vi "CRYO_MASTER_FULL_dev.vi"() -> ()   [LabVIEW 2017] (continued)
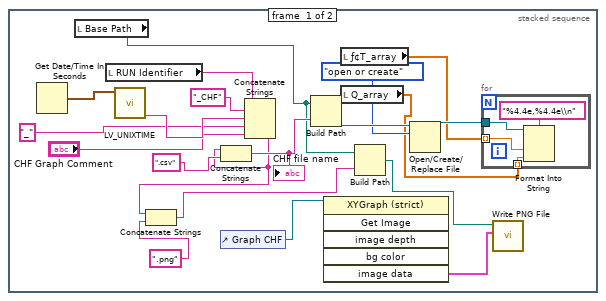
[diagram p3: hidden frame]
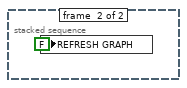
[diagram p5: hidden frame]
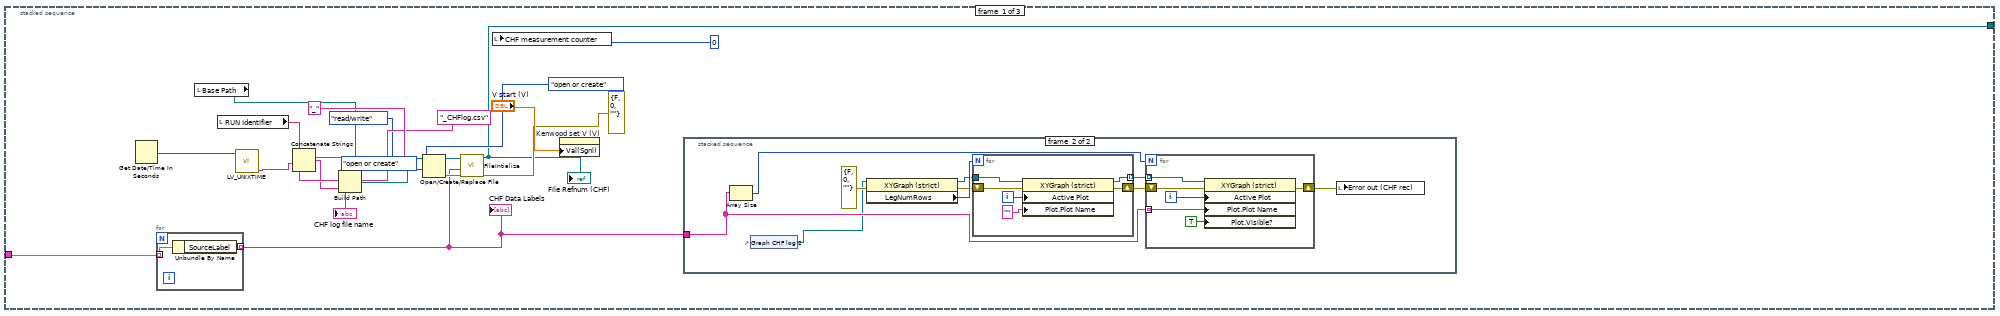
[diagram p7: hidden frame]
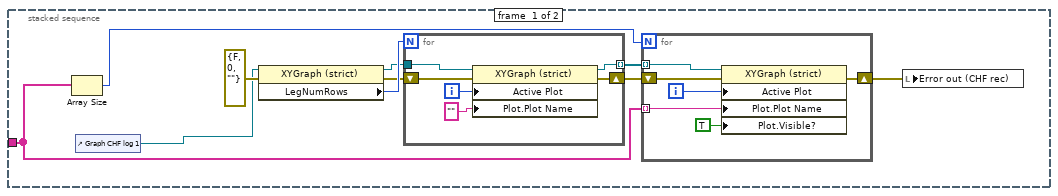
[diagram p8: hidden frame]
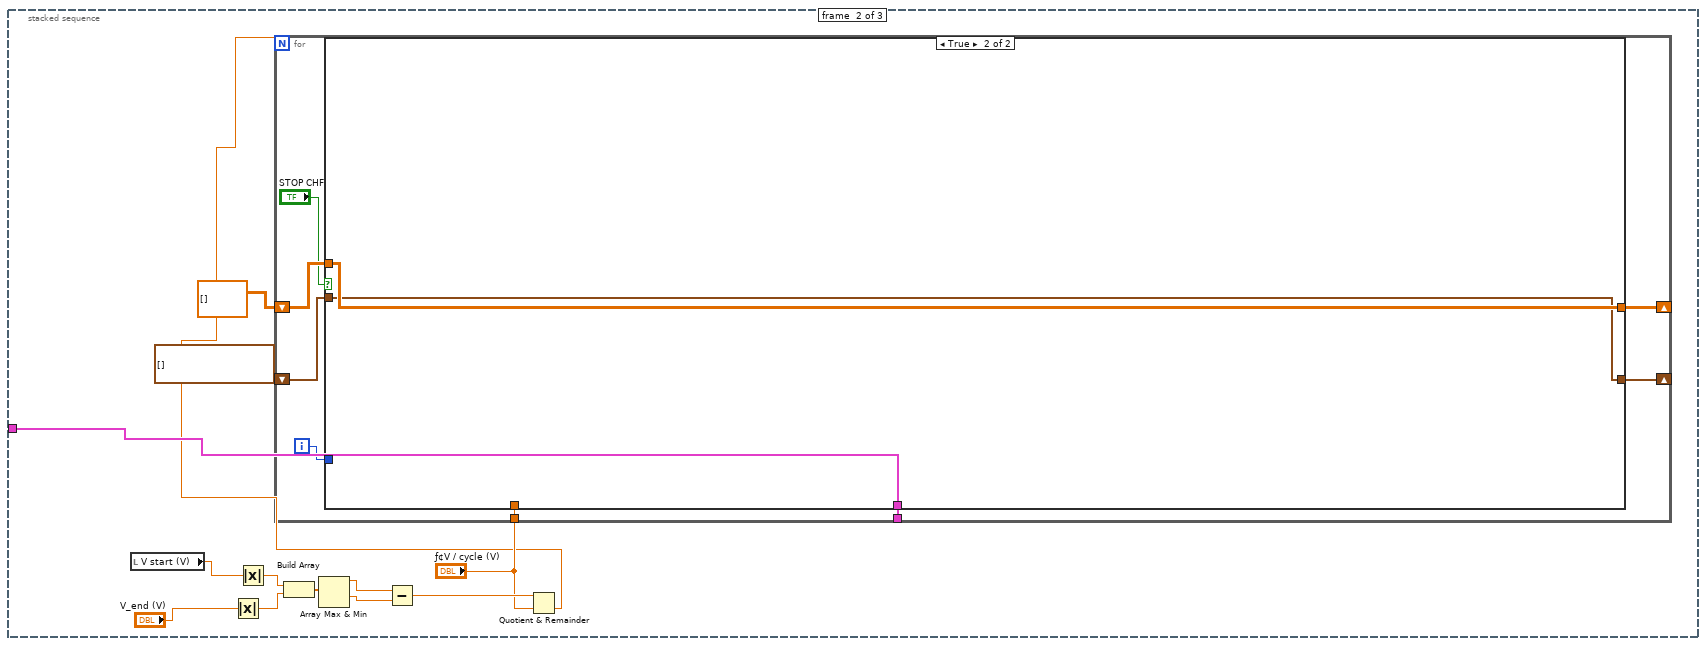
[diagram p9: hidden frame]
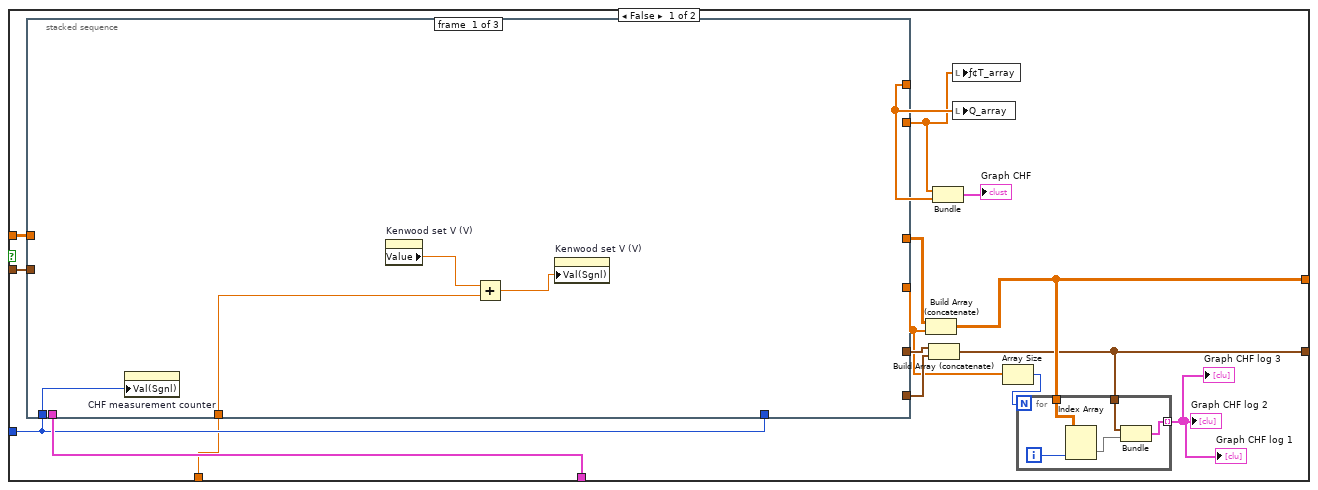
[diagram p10: hidden frame]
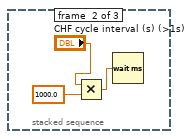
[diagram p11: hidden frame]
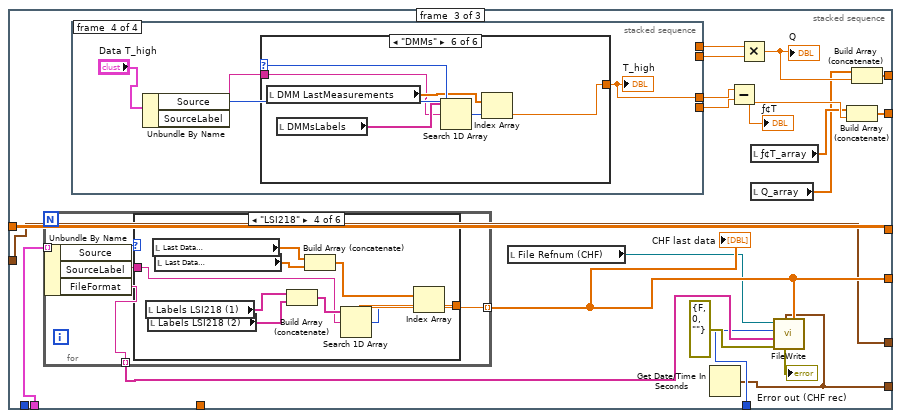
[diagram p12: hidden frame]
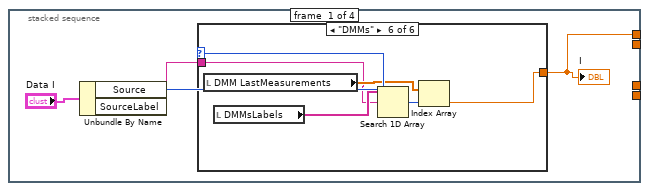
[diagram p13: hidden frame]
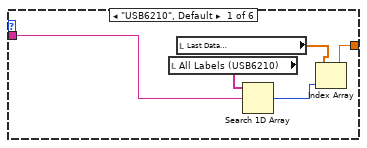
[diagram p14: hidden frame]
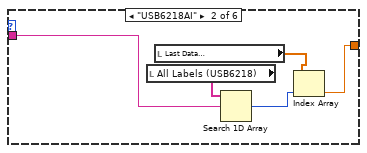
[diagram p15: hidden frame]
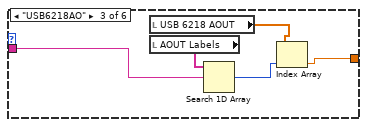
[diagram p16: hidden frame]
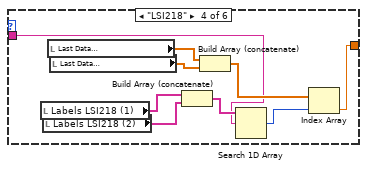
[diagram p17: hidden frame]
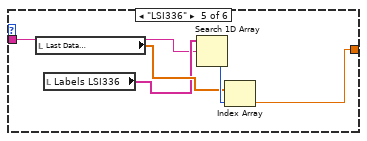
[diagram p18: hidden frame]
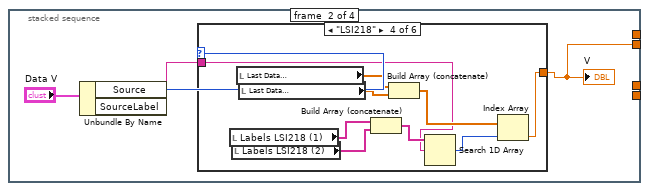
[diagram p19: hidden frame]
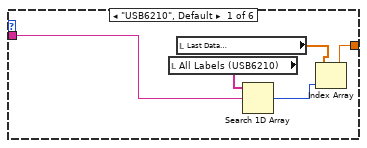
[diagram p20: hidden frame]
    "Cycle #" <- w842
  }
  n1008 = while {
    tunnel: w5 -> [w2128]
    tunnel: w4 -> [w2127]
    stop <- w2129 stop-if-true
    n1009 = Wait (ms)(milliseconds to wait=u32 214) -> ()  [unwired: 1 out]
    n1010 = case shown="True" "RECORD GRAPH" {
      frame False {
      }
      frame True {
        n1011 = stacked-sequence {
          frame #0 {
            n1012 = Get Date/Time In Seconds() -> (seconds since 1Jan1904=w2150:timestamp)
            n1013 = local read "Base Path"() -> (w2135:path)
            n1014 = local read "RUN Identifier"() -> (w2151:string)
            n1015 = call "LV_UNIXTIME.vi"("current time"=w2150) -> ("date/time string"=w2152:string)  [unwired: 9 in, 1 out]
            n1016 = control-ref of="Graph CHF"() -> (w2141:refnum<vi>)
            n1017 = Concatenate Strings(w2151, "_CHF" ("string"), w2152, "_" ("string"), "CHF Graph Comment") -> (w2137:string)
            n1018 = Concatenate Strings(w2137, ".png" ("string")) -> (w2136:string)
            n1019 = Concatenate Strings(w2137, ".csv" ("string")) -> (w2139:string)
            "CHF file name" <- w2139
            n1020 = Build Path(base path=w2135, name or relative path=w2139) -> (appended path=w2146:path)
            n1021 = invoke class="XYGraph (strict)" method="Get Image"(reference=w2141) -> ("image data"=w2133:T23)  [unwired: 5 in, 5 out]
            n1022 = local read "ƒ¢T_array"() -> (w2143:dbl[])
            n1023 = local read "Q_array"() -> (w2142:dbl[])
            n1024 = Build Path(base path=w2135, name or relative path=w2136) -> (appended path=w2134:path)
            n1025 = Open/Create/Replace File(file path (use dialog)=w2146, operation (0:open)=T24."open or create") -> (refnum out=w2144:refnum<file>)  [unwired: 4 in, 2 out]
            n1026 = for {
              tunnel: w2144 -> [w2156]
              tunnel: w2143 -> [w2154] mode=indexing
              tunnel: w2142 -> [w2153] mode=indexing
              n1027 = Format Into String(format string="%4.4e,%4.4e\\n" ("prompt"), initial string=w2156, w2154, w2153) -> ()  [unwired: 1 in, 2 out]
            }
            n1028 = call <vilib>:"Write PNG File.vi"("image data"=w2133, "path to PNG file"=w2134) -> ()  [unwired: 8 in, 2 out]
          }
          frame #1 {
            n1029 = local write "RECORD GRAPH"(FALSE ("RECORD GRAPH")) -> ()
          }
        }
      }
    }
    n1030 = case shown="True" "START CHF" {
      tunnel: "RecordSettings" -> [_ w2161]
      frame False {
      }
      frame True {
        n1031 = stacked-sequence {
          tunnel: [w2165 _ _] -> _
          tunnel: w2161 -> [w2164 w2238 _]
          frame #0 {
            (unwired) T24."open or create" ("operation (0:open)")
            n1032 = Get Date/Time In Seconds() -> (seconds since 1Jan1904=w2177:timestamp)
            n1033 = for {
              tunnel: [w2225] -> w2163 mode=indexing
              tunnel: w2164 -> [w2224] mode=indexing
              n1034 = Unbundle By Name(w2224) -> ("SourceLabel"=w2225:string)
            }
            "CHF Data Labels" <- w2163
            n1035 = local read "Base Path"() -> (w2172:path)
            n1036 = local read "RUN Identifier"() -> (w2176:string)
            n1037 = call "LV_UNIXTIME.vi"("current time"=w2177) -> ("date/time string"=w2175:string)  [unwired: 9 in, 1 out]
            n1038 = Concatenate Strings(w2176, "_" ("string"), w2175, "_CHFlog.csv" ("string")) -> (w2171:string)
            "CHF log file name" <- w2171
            n1039 = Build Path(base path=w2172, name or relative path=w2171) -> (appended path=w2170:path)
            n1040 = Open/Create/Replace File(file path (use dialog)=w2170, error in=errorcluster {"status"=FALSE, "code"=0, "source"=""}, operation (0:open)=T24."open or create", access (0:read/write)=enum16{"read/write", "read-only", "write-only"}."read/write") -> (refnum out=w2168:refnum<file>, error out=w2167:errorcluster)  [unwired: 2 in, 1 out]
            n1041 = call "FileIntialize.vi"("Error In"=w2167, "Labels"=w2163, "refnum in"=w2168) -> ("File Refnum"=w2165:refnum<file>)  [unwired: 7 in, 1 out]
            "File Refnum (CHF)" <- w2165
            n1042 = local write "CHF measurement counter"(0 ("CHF counter")) -> ()
            n1043 = property on="Kenwood set V (V)" class="DigNum (strict)"("Val(Sgnl)"="V start (V)") -> ()  [unwired: 2 in, 2 out]
            n1044 = stacked-sequence {
              tunnel: w2163 -> [w2181 w2204]
              frame #0 {
                n1045 = Array Size(array=w2181) -> (size(s)=w2189:i32)
                n1046 = control-ref of="Graph CHF log 1"() -> (w2182:refnum<vi>)
                n1047 = property class="XYGraph (strict)"(reference=w2182, error in=errorcluster {"status"=FALSE, "code"=0, "source"=""} ("error in (no error)")) -> (reference out=w2184:refnum<vi>, error out=w2186:errorcluster, "LegNumRows"=w2187:u32)
                n1048 = for {
                  N: w2187 -> [_]
                  shift-right: [w2198] -> w2188
                  shift-left: w2186 -> [w2199]
                  tunnel: w2184 -> [w2197]
                  tunnel: [w2196] -> w2183 mode=indexing
                  i -> [w2201]
                  n1049 = property class="XYGraph (strict)"(reference=w2197, error in=w2199, "Active Plot"=w2201, "Plot.Plot Name"="") -> (reference out=w2196:refnum<vi>, error out=w2198:errorcluster)
                }
                n1050 = for {
                  N: w2189 -> [_]
                  shift-right: [w2193] -> w2180
                  shift-left: w2188 -> [w2194]
                  tunnel: w2183 -> [w2191] mode=indexing
                  tunnel: w2181 -> [w2190] mode=indexing
                  i -> [w2195]
                  n1051 = property class="XYGraph (strict)"(reference=w2191, error in=w2194, "Active Plot"=w2195, "Plot.Plot Name"=w2190, "Plot.Visible?"=TRUE ("Plot.Visible")) -> (error out=w2193:errorcluster)  [unwired: 1 out]
                }
                n1052 = local write "Error out (CHF rec)"(w2180) -> ()
              }
              frame #1 {
                n1053 = Array Size(array=w2204) -> (size(s)=w2211:i32)
                n1054 = control-ref of="Graph CHF log 2"() -> (w2203:refnum<vi>)
                n1055 = property class="XYGraph (strict)"(reference=w2203, error in=errorcluster {"status"=FALSE, "code"=0, "source"=""} ("error in (no error)")) -> (reference out=w2206:refnum<vi>, error out=w2208:errorcluster, "LegNumRows"=w2209:u32)
                n1056 = for {
                  N: w2209 -> [_]
                  shift-right: [w2220] -> w2210
                  shift-left: w2208 -> [w2221]
                  tunnel: w2206 -> [w2219]
                  tunnel: [w2218] -> w2205 mode=indexing
                  i -> [w2223]
                  n1057 = property class="XYGraph (strict)"(reference=w2219, error in=w2221, "Active Plot"=w2223, "Plot.Plot Name"="") -> (reference out=w2218:refnum<vi>, error out=w2220:errorcluster)
                }
                n1058 = for {
                  N: w2211 -> [_]
                  shift-right: [w2215] -> w2202
                  shift-left: w2210 -> [w2216]
                  tunnel: w2205 -> [w2213] mode=indexing
                  tunnel: w2204 -> [w2212] mode=indexing
                  i -> [w2217]
                  n1059 = property class="XYGraph (strict)"(reference=w2213, error in=w2216, "Active Plot"=w2217, "Plot.Plot Name"=w2212, "Plot.Visible?"=TRUE ("Plot.Visible")) -> (error out=w2215:errorcluster)  [unwired: 1 out]
                }
                n1060 = local write "Error out (CHF rec)"(w2202) -> ()
              }
            }
          }
          frame #1 {
            n1061 = local read "V start (V)"() -> (w2237:dbl)
            n1062 = Absolute Value(x="V_end (V)") -> (abs(x)=w2234:dbl)
            n1063 = Absolute Value(x=w2237) -> (abs(x)=w2235:dbl)
            n1064 = Build Array(w2235, w2234) -> (w2233:dbl[])
            n1065 = Array Max & Min(array=w2233) -> (max value=w2232:dbl, min value=w2231:dbl)  [unwired: 2 out]
            n1066 = Subtract(x=w2232, y=w2231) -> (x-y=w2230:dbl)
            n1067 = Quotient & Remainder(x=w2230, y="ƒ¢V / cycle (V)") -> (floor(x/y)=w2228:dbl)  [unwired: 1 out]
            n1068 = for {
              N: w2228 -> [_]
              tunnel: w2238 -> [w2246]
              shift-right: [w2242] -> _
              shift-left: dbl[][] [] -> [w2244]
              shift-right: [w2241] -> _
              shift-left: timestamp[] [] -> [w2243]
              tunnel: "ƒ¢V / cycle (V)" -> [w2240]
              i -> [w2245]
              n1069 = case shown="True" "STOP CHF" {
                tunnel: w2246 -> [w2262 _]
                tunnel: w2245 -> [w2261 _]
                tunnel: w2244 -> [w2260 w2487]
                tunnel: w2243 -> [w2256 w2486]
                tunnel: [w2253 w2487] -> w2242
                tunnel: [w2252 w2486] -> w2241
                tunnel: w2240 -> [w2247 _]
                frame False {
                  n1070 = stacked-sequence {
                    tunnel: w2262 -> [_ _ w2294]
                    tunnel: [_ _ w2285] -> w2251
                    tunnel: w2261 -> [_ _ w2284]
                    tunnel: w2261 -> [w2269 _ _]
                    tunnel: [_ _ w2282] -> w2250
                    tunnel: [_ _ w2281] -> w2255
                    tunnel: [_ _ w2280] -> w2259
                    tunnel: w2260 -> [_ _ w2280]
                    tunnel: [_ _ w2279] -> w2258
                    tunnel: w2256 -> [_ _ w2278]
                    tunnel: [_ _ w2278] -> w2257
                    tunnel: w2247 -> [w2268 _ _]
                    frame #0 {
                      n1071 = property on="CHF measurement counter" class="DigNum (strict)"("Val(Sgnl)"=w2269) -> ()  [unwired: 2 in, 2 out]
                      n1072 = property on="Kenwood set V (V)" class="DigNum (strict)"() -> ("Value"=w2271:dbl)  [unwired: 2 in, 2 out]
                      n1073 = Add(x=w2271, y=w2268) -> (x+y=w2270:dbl)
                      n1074 = property on="Kenwood set V (V)" class="DigNum (strict)"("Val(Sgnl)"=w2270) -> ()  [unwired: 2 in, 2 out]
                    }
                    frame #1 {
                      n1075 = Multiply(x="CHF cycle interval (s) (>1s)", y=1000.0) -> (x*y=w2273:dbl)
                      n1076 = Wait (ms)(milliseconds to wait=w2273) -> ()  [unwired: 1 out]
                    }
                    frame #2 {
                      n1077 = for {
                        tunnel: w2294 -> [w2451] mode=indexing
                        tunnel: [w2449] -> w2281 mode=indexing
                        tunnel: [w2447] -> w2292 mode=indexing
                        n1078 = Unbundle By Name(w2451) -> ("Source"=w2450:T36, "SourceLabel"=w2448:string, "FileFormat"=w2447:string)
                        n1079 = case shown="\"LSI218\"" w2450 {
                          tunnel: [w2452 w2457 w2462 w2468 w2476 w2481] -> w2449
                          tunnel: w2448 -> [w2453 w2459 w2464 w2467 w2477 w2485]
                          frame "USB6210", Default {
                            n1080 = local read "All Labels (USB6210)"() -> (w2455:string[])
                            n1081 = local read "Last Data \n(USB6210)"() -> (w2456:dbl[])
                            n1082 = Search 1D Array(1D array=w2455, element=w2453) -> (index of element=w2454:i32)  [unwired: 1 in]
                            n1083 = Index Array(array=w2456, index=w2454) -> (element=w2452:dbl)
                          }
                          frame "USB6218AI" {
                            n1084 = local read "All Labels (USB6218)"() -> (w2460:string[])
                            n1085 = local read "Last Data \n(USB6218)"() -> (w2461:dbl[])
                            n1086 = Search 1D Array(1D array=w2460, element=w2459) -> (index of element=w2458:i32)  [unwired: 1 in]
                            n1087 = Index Array(array=w2461, index=w2458) -> (element=w2457:dbl)
                          }
                          frame "USB6218AO" {
                            n1088 = local read "USB 6218 AOUT"() -> (w2466:dbl[])
                            n1089 = local read "AOUT Labels"() -> (w2465:string[])
                            n1090 = Search 1D Array(1D array=w2465, element=w2464) -> (index of element=w2463:i32)  [unwired: 1 in]
                            n1091 = Index Array(array=w2466, index=w2463) -> (element=w2462:dbl)
                          }
                          frame "LSI218" {
                            n1092 = local read "Labels LSI218 (1)"() -> (w2471:string[])
                            n1093 = local read "Labels LSI218 (2)"() -> (w2470:string[])
                            n1094 = local read "Last Data \nLSI218 (1)"() -> (w2474:dbl[])
                            n1095 = local read "Last Data \nLSI218 (2)"() -> (w2473:dbl[])
                            n1096 = Build Array (concatenate)(w2471, w2470) -> (w2469:string[])
                            n1097 = Build Array (concatenate)(w2474, w2473) -> (w2472:dbl[])
                            n1098 = Search 1D Array(1D array=w2469, element=w2467) -> (index of element=w2475:i32)  [unwired: 1 in]
                            n1099 = Index Array(array=w2472, index=w2475) -> (element=w2468:dbl)
                          }
                          frame "LSI336" {
                            n1100 = local read "Last Data \nLSI336"() -> (w2479:dbl[])
                            n1101 = local read "Labels LSI336"() -> (w2480:string[])
                            n1102 = Search 1D Array(1D array=w2480, element=w2477) -> (index of element=w2478:i32)  [unwired: 1 in]
                            n1103 = Index Array(array=w2479, index=w2478) -> (element=w2476:dbl)
                          }
                          frame "DMMs" {
                            n1104 = local read "DMM LastMeasurements"() -> (w2482:dbl[])
                            n1105 = local read "DMMsLabels"() -> (w2484:string[])
                            n1106 = Search 1D Array(1D array=w2484, element=w2485) -> (index of element=w2483:i32)  [unwired: 1 in]
                            n1107 = Index Array(array=w2482, index=w2483) -> (element=w2481:dbl)
                          }
                        }
                      }
                      "CHF last data" <- w2281
                      n1108 = stacked-sequence {
                        tunnel: [w2295 _ _ _] -> w2290
                        tunnel: [_ w2333 _ _] -> w2289
                        tunnel: [_ _ _ w2409] -> w2288
                        tunnel: [_ _ w2371 _] -> w2287
                        frame #0 {
                          n1109 = Unbundle By Name("Data I") -> ("Source"=w2297:T36, "SourceLabel"=w2296:string)
                          n1110 = case shown="\"DMMs\"" w2297 {
                            tunnel: w2296 -> [w2300 w2305 w2310 w2315 w2324 w2329]
                            tunnel: [w2299 w2304 w2309 w2314 w2323 w2328] -> w2295
                            frame "USB6210", Default {
                              n1111 = local read "All Labels (USB6210)"() -> (w2302:string[])
                              n1112 = local read "Last Data \n(USB6210)"() -> (w2301:dbl[])
                              n1113 = Search 1D Array(1D array=w2302, element=w2300) -> (index of element=w2303:i32)  [unwired: 1 in]
                              n1114 = Index Array(array=w2301, index=w2303) -> (element=w2299:dbl)
                            }
                            frame "USB6218AI" {
                              n1115 = local read "All Labels (USB6218)"() -> (w2307:string[])
                              n1116 = local read "Last Data \n(USB6218)"() -> (w2306:dbl[])
                              n1117 = Search 1D Array(1D array=w2307, element=w2305) -> (index of element=w2308:i32)  [unwired: 1 in]
                              n1118 = Index Array(array=w2306, index=w2308) -> (element=w2304:dbl)
                            }
                            frame "USB6218AO" {
                              n1119 = local read "USB 6218 AOUT"() -> (w2311:dbl[])
                              n1120 = local read "AOUT Labels"() -> (w2312:string[])
                              n1121 = Search 1D Array(1D array=w2312, element=w2310) -> (index of element=w2313:i32)  [unwired: 1 in]
                              n1122 = Index Array(array=w2311, index=w2313) -> (element=w2309:dbl)
                            }
                            frame "LSI218" {
                              n1123 = local read "Labels LSI218 (1)"() -> (w2320:string[])
                              n1124 = local read "Labels LSI218 (2)"() -> (w2321:string[])
                              n1125 = local read "Last Data \nLSI218 (1)"() -> (w2317:dbl[])
                              n1126 = local read "Last Data \nLSI218 (2)"() -> (w2318:dbl[])
                              n1127 = Build Array (concatenate)(w2320, w2321) -> (w2322:string[])
                              n1128 = Build Array (concatenate)(w2317, w2318) -> (w2319:dbl[])
                              n1129 = Search 1D Array(1D array=w2322, element=w2315) -> (index of element=w2316:i32)  [unwired: 1 in]
                              n1130 = Index Array(array=w2319, index=w2316) -> (element=w2314:dbl)
                            }
                            frame "LSI336" {
                              n1131 = local read "Last Data \nLSI336"() -> (w2326:dbl[])
                              n1132 = local read "Labels LSI336"() -> (w2325:string[])
                              n1133 = Search 1D Array(1D array=w2325, element=w2324) -> (index of element=w2327:i32)  [unwired: 1 in]
                              n1134 = Index Array(array=w2326, index=w2327) -> (element=w2323:dbl)
                            }
                            frame "DMMs" {
                              n1135 = local read "DMM LastMeasurements"() -> (w2332:dbl[])
                              n1136 = local read "DMMsLabels"() -> (w2330:string[])
                              n1137 = Search 1D Array(1D array=w2330, element=w2329) -> (index of element=w2331:i32)  [unwired: 1 in]
                              n1138 = Index Array(array=w2332, index=w2331) -> (element=w2328:dbl)
                            }
                          }
                          "I" <- w2295
                        }
                        frame #1 {
                          n1139 = Unbundle By Name("Data V") -> ("Source"=w2336:T36, "SourceLabel"=w2335:string)
                          n1140 = case shown="\"LSI218\"" w2336 {
                            tunnel: w2335 -> [w2338 w2343 w2348 w2353 w2362 w2367]
                            tunnel: [w2337 w2342 w2347 w2352 w2361 w2366] -> w2333
                            frame "USB6210", Default {
                              n1141 = local read "All Labels (USB6210)"() -> (w2340:string[])
                              n1142 = local read "Last Data \n(USB6210)"() -> (w2339:dbl[])
                              n1143 = Search 1D Array(1D array=w2340, element=w2338) -> (index of element=w2341:i32)  [unwired: 1 in]
                              n1144 = Index Array(array=w2339, index=w2341) -> (element=w2337:dbl)
                            }
                            frame "USB6218AI" {
                              n1145 = local read "All Labels (USB6218)"() -> (w2345:string[])
                              n1146 = local read "Last Data \n(USB6218)"() -> (w2344:dbl[])
                              n1147 = Search 1D Array(1D array=w2345, element=w2343) -> (index of element=w2346:i32)  [unwired: 1 in]
                              n1148 = Index Array(array=w2344, index=w2346) -> (element=w2342:dbl)
                            }
                            frame "USB6218AO" {
                              n1149 = local read "USB 6218 AOUT"() -> (w2349:dbl[])
                              n1150 = local read "AOUT Labels"() -> (w2350:string[])
                              n1151 = Search 1D Array(1D array=w2350, element=w2348) -> (index of element=w2351:i32)  [unwired: 1 in]
                              n1152 = Index Array(array=w2349, index=w2351) -> (element=w2347:dbl)
                            }
                            frame "LSI218" {
                              n1153 = local read "Labels LSI218 (1)"() -> (w2358:string[])
                              n1154 = local read "Labels LSI218 (2)"() -> (w2359:string[])
                              n1155 = local read "Last Data \nLSI218 (1)"() -> (w2355:dbl[])
                              n1156 = local read "Last Data \nLSI218 (2)"() -> (w2356:dbl[])
                              n1157 = Build Array (concatenate)(w2358, w2359) -> (w2360:string[])
                              n1158 = Build Array (concatenate)(w2355, w2356) -> (w2357:dbl[])
                              n1159 = Search 1D Array(1D array=w2360, element=w2353) -> (index of element=w2354:i32)  [unwired: 1 in]
                              n1160 = Index Array(array=w2357, index=w2354) -> (element=w2352:dbl)
                            }
                            frame "LSI336" {
                              n1161 = local read "Last Data \nLSI336"() -> (w2364:dbl[])
                              n1162 = local read "Labels LSI336"() -> (w2363:string[])
                              n1163 = Search 1D Array(1D array=w2363, element=w2362) -> (index of element=w2365:i32)  [unwired: 1 in]
                              n1164 = Index Array(array=w2364, index=w2365) -> (element=w2361:dbl)
                            }
                            frame "DMMs" {
                              n1165 = local read "DMM LastMeasurements"() -> (w2370:dbl[])
                              n1166 = local read "DMMsLabels"() -> (w2368:string[])
                              n1167 = Search 1D Array(1D array=w2368, element=w2367) -> (index of element=w2369:i32)  [unwired: 1 in]
                              n1168 = Index Array(array=w2370, index=w2369) -> (element=w2366:dbl)
                            }
                          }
                          "V" <- w2333
                        }
                        frame #2 {
                          n1169 = Unbundle By Name("Data T_low") -> ("Source"=w2374:T36, "SourceLabel"=w2373:string)
                          n1170 = case shown="\"DMMs\"" w2374 {
                            tunnel: w2373 -> [w2376 w2381 w2386 w2391 w2400 w2405]
                            tunnel: [w2375 w2380 w2385 w2390 w2399 w2404] -> w2371
                            frame "USB6210", Default {
                              n1171 = local read "All Labels (USB6210)"() -> (w2378:string[])
                              n1172 = local read "Last Data \n(USB6210)"() -> (w2377:dbl[])
                              n1173 = Search 1D Array(1D array=w2378, element=w2376) -> (index of element=w2379:i32)  [unwired: 1 in]
                              n1174 = Index Array(array=w2377, index=w2379) -> (element=w2375:dbl)
                            }
                            frame "USB6218AI" {
                              n1175 = local read "All Labels (USB6218)"() -> (w2383:string[])
                              n1176 = local read "Last Data \n(USB6218)"() -> (w2382:dbl[])
                              n1177 = Search 1D Array(1D array=w2383, element=w2381) -> (index of element=w2384:i32)  [unwired: 1 in]
                              n1178 = Index Array(array=w2382, index=w2384) -> (element=w2380:dbl)
                            }
                            frame "USB6218AO" {
                              n1179 = local read "USB 6218 AOUT"() -> (w2387:dbl[])
                              n1180 = local read "AOUT Labels"() -> (w2388:string[])
                              n1181 = Search 1D Array(1D array=w2388, element=w2386) -> (index of element=w2389:i32)  [unwired: 1 in]
                              n1182 = Index Array(array=w2387, index=w2389) -> (element=w2385:dbl)
                            }
                            frame "LSI218" {
                              n1183 = local read "Labels LSI218 (1)"() -> (w2396:string[])
                              n1184 = local read "Labels LSI218 (2)"() -> (w2397:string[])
                              n1185 = local read "Last Data \nLSI218 (1)"() -> (w2393:dbl[])
                              n1186 = local read "Last Data \nLSI218 (2)"() -> (w2394:dbl[])
                              n1187 = Build Array (concatenate)(w2396, w2397) -> (w2398:string[])
                              n1188 = Build Array (concatenate)(w2393, w2394) -> (w2395:dbl[])
                              n1189 = Search 1D Array(1D array=w2398, element=w2391) -> (index of element=w2392:i32)  [unwired: 1 in]
                              n1190 = Index Array(array=w2395, index=w2392) -> (element=w2390:dbl)
                            }
                            frame "LSI336" {
                              n1191 = local read "Last Data \nLSI336"() -> (w2402:dbl[])
                              n1192 = local read "Labels LSI336"() -> (w2401:string[])
                              n1193 = Search 1D Array(1D array=w2401, element=w2400) -> (index of element=w2403:i32)  [unwired: 1 in]
                              n1194 = Index Array(array=w2402, index=w2403) -> (element=w2399:dbl)
                            }
                            frame "DMMs" {
                              n1195 = local read "DMM LastMeasurements"() -> (w2408:dbl[])
                              n1196 = local read "DMMsLabels"() -> (w2406:string[])
                              n1197 = Search 1D Array(1D array=w2406, element=w2405) -> (index of element=w2407:i32)  [unwired: 1 in]
                              n1198 = Index Array(array=w2408, index=w2407) -> (element=w2404:dbl)
                            }
                          }
                          "T_low" <- w2371
                        }
                        frame #3 {
                          n1199 = Unbundle By Name("Data T_high") -> ("Source"=w2412:T36, "SourceLabel"=w2411:string)
                          n1200 = case shown="\"DMMs\"" w2412 {
                            tunnel: w2411 -> [w2414 w2419 w2424 w2429 w2438 w2443]
                            tunnel: [w2413 w2418 w2423 w2428 w2437 w2442] -> w2409
                            frame "USB6210", Default {
                              n1201 = local read "All Labels (USB6210)"() -> (w2416:string[])
                              n1202 = local read "Last Data \n(USB6210)"() -> (w2415:dbl[])
                              n1203 = Search 1D Array(1D array=w2416, element=w2414) -> (index of element=w2417:i32)  [unwired: 1 in]
                              n1204 = Index Array(array=w2415, index=w2417) -> (element=w2413:dbl)
                            }
                            frame "USB6218AI" {
                              n1205 = local read "All Labels (USB6218)"() -> (w2421:string[])
                              n1206 = local read "Last Data \n(USB6218)"() -> (w2420:dbl[])
                              n1207 = Search 1D Array(1D array=w2421, element=w2419) -> (index of element=w2422:i32)  [unwired: 1 in]
                              n1208 = Index Array(array=w2420, index=w2422) -> (element=w2418:dbl)
                            }
                            frame "USB6218AO" {
                              n1209 = local read "USB 6218 AOUT"() -> (w2425:dbl[])
                              n1210 = local read "AOUT Labels"() -> (w2426:string[])
                              n1211 = Search 1D Array(1D array=w2426, element=w2424) -> (index of element=w2427:i32)  [unwired: 1 in]
                              n1212 = Index Array(array=w2425, index=w2427) -> (element=w2423:dbl)
                            }
                            frame "LSI218" {
                              n1213 = local read "Labels LSI218 (1)"() -> (w2434:string[])
                              n1214 = local read "Labels LSI218 (2)"() -> (w2435:string[])
                              n1215 = local read "Last Data \nLSI218 (1)"() -> (w2431:dbl[])
                              n1216 = local read "Last Data \nLSI218 (2)"() -> (w2432:dbl[])
                              n1217 = Build Array (concatenate)(w2434, w2435) -> (w2436:string[])
                              n1218 = Build Array (concatenate)(w2431, w2432) -> (w2433:dbl[])
                              n1219 = Search 1D Array(1D array=w2436, element=w2429) -> (index of element=w2430:i32)  [unwired: 1 in]
                              n1220 = Index Array(array=w2433, index=w2430) -> (element=w2428:dbl)
                            }
                            frame "LSI336" {
                              n1221 = local read "Last Data \nLSI336"() -> (w2440:dbl[])
                              n1222 = local read "Labels LSI336"() -> (w2439:string[])
                              n1223 = Search 1D Array(1D array=w2439, element=w2438) -> (index of element=w2441:i32)  [unwired: 1 in]
                              n1224 = Index Array(array=w2440, index=w2441) -> (element=w2437:dbl)
                            }
                            frame "DMMs" {
                              n1225 = local read "DMM LastMeasurements"() -> (w2446:dbl[])
                              n1226 = local read "DMMsLabels"() -> (w2444:string[])
                              n1227 = Search 1D Array(1D array=w2444, element=w2443) -> (index of element=w2445:i32)  [unwired: 1 in]
                              n1228 = Index Array(array=w2446, index=w2445) -> (element=w2442:dbl)
                            }
                          }
                          "T_high" <- w2409
                        }
                      }
                      n1229 = local read "File Refnum (CHF)"() -> (w2275:refnum<file>)
                      n1230 = Get Date/Time In Seconds() -> (seconds since 1Jan1904=w2279:timestamp)
                      n1231 = Subtract(x=w2288, y=w2287) -> (x-y=w2283:dbl)
                      "ƒ¢T" <- w2283
                      n1232 = Multiply(x=w2290, y=w2289) -> (x*y=w2286:dbl)
                      "Q" <- w2286
                      n1233 = local read "ƒ¢T_array"() -> (w2277:dbl[])
                      n1234 = local read "Q_array"() -> (w2276:dbl[])
                      n1235 = call "FileWrite.vi"("DataArray"=w2281, "Time Stamp"=w2279, "Error In"=errorcluster {"status"=FALSE, "code"=0, "source"=""}, "FileFormat"=w2292, "Index"=w2284, "refnum in"=w2275) -> ("Error Out"=→"Error out (CHF rec)":errorcluster)  [unwired: 4 in, 1 out]
                      n1236 = Build Array (concatenate)(w2277, w2283) -> (w2282:dbl[])
                      n1237 = Build Array (concatenate)(w2276, w2286) -> (w2285:dbl[])
                    }
                  }
                  n1238 = Build Array (concatenate)(w2259, w2255) -> (w2253:dbl[][])
                  n1239 = Build Array (concatenate)(w2257, w2258) -> (w2252:timestamp[])
                  n1240 = Bundle(w2250, w2251) -> (→"Graph CHF":cluster{dbl[], dbl[]})  [unwired: 1 in]
                  n1241 = local write "ƒ¢T_array"(w2250) -> ()
                  n1242 = local write "Q_array"(w2251) -> ()
                  n1243 = Array Size(array=w2255) -> (size(s)=w2254:i32)
                  n1244 = for {
                    N: w2254 -> [_]
                    tunnel: w2253 -> [w2267]
                    tunnel: w2252 -> [w2265]
                    tunnel: [w2263] -> w2248 mode=indexing
                    i -> [w2266]
                    n1245 = Index Array(array=w2267, index (col)=w2266) -> (element=w2264:dbl[])  [unwired: 1 in]
                    n1246 = Bundle(w2265, w2264) -> (w2263:cluster{timestamp[], dbl[]})  [unwired: 1 in]
                  }
                  "Graph CHF log 2" <- w2248
                  "Graph CHF log 1" <- w2248
                  "Graph CHF log 3" <- w2248
                }
                frame True {
                }
              }
            }
          }
          frame #2 {
            n1247 = local write "CHF measurement counter"(0 ("CHF counter")) -> ()
            n1248 = local write "START CHF"(FALSE ("START CHF")) -> ()
            n1249 = local write "STOP CHF"(FALSE ("STOP CHF")) -> ()
          }
        }
      }
    }
    n1250 = case shown="True" "REFRESH GRAPH" {
      frame False {
      }
      frame True {
        n1251 = stacked-sequence {
          frame #0 {
            w2159 = dbl[] [] ("ƒ¢T_array")
            n1252 = local write "ƒ¢T_array"(w2159) -> ()
            n1253 = local write "Q_array"(w2159) -> ()
            n1254 = Bundle("ƒ¢T_array"=w2159, "ƒ¢T_array"=w2159) -> (w2158:cluster{"ƒ¢T_array":dbl[], "ƒ¢T_array":dbl[]})  [unwired: 1 in]
            n1255 = local write "Graph CHF"(w2158) -> ()
          }
          frame #1 {
            n1256 = local write "REFRESH GRAPH"(FALSE ("REFRESH GRAPH")) -> ()
          }
        }
      }
    }
    n1257 = Get Notifier Status(notifier=w2128, error in (no error)=w2127) -> (current notification=w2129:bool)  [unwired: 4 out]
  }
  n1258 = while {
    shift-right: [w2500] -> w8
    shift-left: refnum<class "DMMsData.lvclass"> refnum ("DMMsData.lvclass") -> [w2499]
    shift-right: [w2498] -> w7
    shift-left: errorcluster {"status"=FALSE, "code"=0, "source"=""} ("error in (no error)") -> [w2491]
    tunnel: w5 -> [w2496]
    tunnel: w4 -> [w2495]
    tunnel: [w2494] -> w11
    i -> [w2497]
    stop <- w2493 stop-if-true
    n1259 = Equal?(x=w2497, y=0) -> (x = y?=w2501:bool)
    n1260 = Wait (ms)(milliseconds to wait="Measurement Interval DMMs (ms)") -> ()  [unwired: 1 out]
    n1261 = case shown="True" "Measure DMMs?" {
      tunnel: w2501 -> [_ w2512]
      tunnel: [w2505 w2510] -> w2500
      tunnel: w2499 -> [w2505 w2509]
      tunnel: w2491 -> [w2504 w2508]
      tunnel: [w2504 w2507] -> w2498
      tunnel: w2497 -> [_ w2506]
      frame False {
      }
      frame True {
        n1262 = Or(x="Initialize (DMMs)", y=w2512) -> (x .or. y?=w2511:bool)
        n1263 = case shown="True" w2511 {
          tunnel: w2509 -> [w2543 w2579]
          tunnel: [w2540 w2578] -> w2510
          tunnel: w2508 -> [w2542 w2575]
          tunnel: [w2541 w2572] -> w2507
          tunnel: w2506 -> [w2539 _]
          frame False {
            n1264 = local read "VariableSources"() -> (w2532:T11)
            n1265 = for {
              tunnel: w2532 -> [w2546] mode=indexing
              tunnel: [w2545] -> w2531 mode=indexing
              tunnel: [w2544] -> w2530 mode=indexing
              n1266 = case shown="\"LSI218\"" w2546 {
                tunnel: [w2548 w2550 w2552 w2553 w2559] -> w2545
                tunnel: [w2547 w2549 w2551 w2554 w2560] -> w2544
                frame "USB6210" {
                  n1267 = local read "All Labels (USB6210)"() -> (w2548:string[])
                  n1268 = local read "Last Data \n(USB6210)"() -> (w2547:dbl[])
                }
                frame "USB6218AI" {
                  n1269 = local read "Last Data \n(USB6218)"() -> (w2549:dbl[])
                  n1270 = local read "All Labels (USB6218)"() -> (w2550:string[])
                }
                frame "USB6218AO" {
                  n1271 = local read "USB 6218 AOUT"() -> (w2551:dbl[])
                  n1272 = local read "AOUT Labels"() -> (w2552:string[])
                }
                frame "LSI218" {
                  n1273 = local read "Last Data \nLSI218 (2)"() -> (w2555:dbl[])
                  n1274 = local read "Last Data \nLSI218 (1)"() -> (w2556:dbl[])
                  n1275 = local read "Labels LSI218 (2)"() -> (w2558:string[])
                  n1276 = local read "Labels LSI218 (1)"() -> (w2557:string[])
                  n1277 = Build Array (concatenate)(w2556, w2555) -> (w2554:dbl[])
                  n1278 = Build Array (concatenate)(w2557, w2558) -> (w2553:string[])
                }
                frame "LSI336" {
                  n1279 = local read "Last Data \nLSI336"() -> (w2560:dbl[])
                  n1280 = local read "Labels LSI336"() -> (w2559:string[])
                }
              }
            }
            n1281 = local read "DMMsConfig (variables)"() -> (w2524:T12)
            n1282 = local read "DMMsConfig"() -> (w2536:T13)
            n1283 = call-dynamic "DMMs_measure.vi"("DMMsData in"=w2543, "Sample #"="Sample #", "MeasurementIndex"=w2539, "SourceDataLabels"=w2531, "error in (no error)"=w2542, "SourceDataArray"=w2530) -> ("TimeArray"=w2538:timestamp[], "DMMsData out"=w2540:refnum<class "DMMsData.lvclass">, "LastData"=w2518:dbl[], "DataArray"=w2535:dbl[][], "DeviceActive?"=→"Active?":bool[], "error out"=w2541:errorcluster)  [unwired: 4 in]
            "DMM LastMeasurements" <- w2518
            n1284 = Array Size(array=w2524) -> (size(s)=w2522:i32)
            n1285 = Array Size(array=w2536) -> (size(s)=w2523:i32)
            n1286 = Add(x=w2523, y=w2522) -> (x+y=w2521:i32)
            n1287 = for {
              N: w2521 -> [_]
              tunnel: w2538 -> [w2563]
              tunnel: w2535 -> [w2567]
              shift-right: [w2561] -> w2520
              shift-left: T4 [] -> [w2562]
              i -> [w2566]
              n1288 = Index Array(array=w2567, index (col)=w2566) -> (element=w2565:dbl[])  [unwired: 1 in]
              n1289 = Bundle("TimeArray"=w2563, "DataArray"=w2565) -> (w2564:T35)  [unwired: 1 in]
              n1290 = Build Array (concatenate)(w2562, w2564) -> (w2561:T4)
            }
            "Graph DMMs 2" <- w2520
            "Graph DMMs 1" <- w2520
            "Graph DMMs 3" <- w2520
            n1291 = Index Array(array=w2518, index #1="index T_2", index #2="index T_ 1") -> (element #1=w2517:dbl, element #2=w2514:dbl)
            n1292 = Index Array(array=w2518, index #1="index V", index #2="index I") -> (element #1=w2527:dbl, element #2=w2526:dbl)
            n1293 = Subtract(x=w2517, y=w2514) -> (x-y=→"ƒ¢T=T_2 -T_1":dbl)
            n1294 = Multiply(x=w2527, y=w2526) -> (x*y=→"Q = I *V":dbl)
          }
          frame True {
            n1295 = local write "Initialize (DMMs)"(FALSE ("Initialize 2")) -> ()
            n1296 = local read "RUN Identifier"() -> (w2570:string)
            n1297 = local read "Base Path"() -> (w2576:path)
            n1298 = call-dynamic "DMMs_initialize.vi"("DMMsConfig (variables)"="DMMsConfig (variables)", "DMMsConfig"="DMMsConfig", "InstName"="InstName DMMs", "error in (no error)"=w2575, "base path"=w2576, "RunIdentifier"=w2570, "DMMsData in"=w2579) -> ("error out"=w2572:errorcluster, "DMMsLabels"=w2573:string[], "FileName"=→"DMMFileName":string, "DMMsData out"=w2578:refnum<class "DMMsData.lvclass">, "VariableSources"=→"VariableSources":T11)
            "DMMsLabels" <- w2573
            n1299 = stacked-sequence {
              tunnel: w2573 -> [w2581 w2604 w2627]
              frame #0 {
                n1300 = Array Size(array=w2581) -> (size(s)=w2590:i32)
                n1301 = control-ref of="Graph DMMs 1"() -> (w2587:refnum<vi>)
                n1302 = property class="XYGraph (strict)"(reference=w2587, error in=errorcluster {"status"=FALSE, "code"=0, "source"=""} ("error in (no error)")) -> (reference out=w2583:refnum<vi>, error out=w2586:errorcluster, "LegNumRows"=w2588:u32)
                n1303 = for {
                  N: w2588 -> [_]
                  shift-right: [w2599] -> w2589
                  shift-left: w2586 -> [w2600]
                  tunnel: w2583 -> [w2598]
                  tunnel: [w2597] -> w2582 mode=indexing
                  i -> [w2602]
                  n1304 = property class="XYGraph (strict)"(reference=w2598, error in=w2600, "Active Plot"=w2602, "Plot.Plot Name"="") -> (reference out=w2597:refnum<vi>, error out=w2599:errorcluster)
                }
                n1305 = for {
                  N: w2590 -> [_]
                  shift-right: [w2594] -> w2584
                  shift-left: w2589 -> [w2595]
                  tunnel: w2582 -> [w2592] mode=indexing
                  tunnel: w2581 -> [w2591] mode=indexing
                  i -> [w2596]
                  n1306 = property class="XYGraph (strict)"(reference=w2592, error in=w2595, "Active Plot"=w2596, "Plot.Plot Name"=w2591, "Plot.Visible?"=TRUE ("Plot.Visible")) -> (error out=w2594:errorcluster)  [unwired: 1 out]
                }
                "error out (DMM graphs)" <- w2584
              }
              frame #1 {
                n1307 = Array Size(array=w2604) -> (size(s)=w2612:i32)
                n1308 = control-ref of="Graph DMMs 2"() -> (w2607:refnum<vi>)
                n1309 = property class="XYGraph (strict)"(reference=w2607, error in=errorcluster {"status"=FALSE, "code"=0, "source"=""} ("error in (no error)")) -> (reference out=w2606:refnum<vi>, error out=w2609:errorcluster, "LegNumRows"=w2610:u32)
                n1310 = for {
                  N: w2610 -> [_]
                  shift-right: [w2621] -> w2611
                  shift-left: w2609 -> [w2622]
                  tunnel: w2606 -> [w2620]
                  tunnel: [w2619] -> w2605 mode=indexing
                  i -> [w2624]
                  n1311 = property class="XYGraph (strict)"(reference=w2620, error in=w2622, "Active Plot"=w2624, "Plot.Plot Name"="") -> (reference out=w2619:refnum<vi>, error out=w2621:errorcluster)
                }
                n1312 = for {
                  N: w2612 -> [_]
                  shift-right: [w2616] -> w2603
                  shift-left: w2611 -> [w2617]
                  tunnel: w2605 -> [w2614] mode=indexing
                  tunnel: w2604 -> [w2613] mode=indexing
                  i -> [w2618]
                  n1313 = property class="XYGraph (strict)"(reference=w2614, error in=w2617, "Active Plot"=w2618, "Plot.Plot Name"=w2613, "Plot.Visible?"=TRUE ("Plot.Visible")) -> (error out=w2616:errorcluster)  [unwired: 1 out]
                }
                n1314 = local write "error out (DMM graphs)"(w2603) -> ()
              }
              frame #2 {
                n1315 = Array Size(array=w2627) -> (size(s)=w2634:i32)
                n1316 = control-ref of="Graph DMMs 3"() -> (w2625:refnum<vi>)
                n1317 = property class="XYGraph (strict)"(reference=w2625, error in=errorcluster {"status"=FALSE, "code"=0, "source"=""} ("error in (no error)")) -> (reference out=w2629:refnum<vi>, error out=w2631:errorcluster, "LegNumRows"=w2632:u32)
                n1318 = for {
                  N: w2632 -> [_]
                  shift-right: [w2643] -> w2633
                  shift-left: w2631 -> [w2644]
                  tunnel: w2629 -> [w2642]
                  tunnel: [w2641] -> w2628 mode=indexing
                  i -> [w2646]
                  n1319 = property class="XYGraph (strict)"(reference=w2642, error in=w2644, "Active Plot"=w2646, "Plot.Plot Name"="") -> (reference out=w2641:refnum<vi>, error out=w2643:errorcluster)
                }
                n1320 = for {
                  N: w2634 -> [_]
                  shift-right: [w2638] -> w2626
                  shift-left: w2633 -> [w2639]
                  tunnel: w2628 -> [w2636] mode=indexing
                  tunnel: w2627 -> [w2635] mode=indexing
                  i -> [w2640]
                  n1321 = property class="XYGraph (strict)"(reference=w2636, error in=w2639, "Active Plot"=w2640, "Plot.Plot Name"=w2635, "Plot.Visible?"=TRUE ("Plot.Visible")) -> (error out=w2638:errorcluster)  [unwired: 1 out]
                }
                n1322 = local write "error out (DMM graphs)"(w2626) -> ()
              }
            }
          }
        }
        "error out (DMMs)" <- w2507
      }
    }
    n1323 = Get Notifier Status(notifier=w2496, error in (no error)=w2495) -> (current notification=w2493:bool, error out=w2494:errorcluster)  [unwired: 3 out]
    "cycle # (DMMs)" <- w2497
  }
  n1324 = call-dynamic "USBData_terminate.vi"("error in (no error)"=w24, "USBData in"=w25) -> ("error out"=w26:errorcluster)  [unwired: 8 in, 1 out]
  n1325 = local write "error out (USB6210)"(w26) -> ()
  n1326 = call-dynamic "DMMs_terminate.vi"("error in (no error)"=w7, "DMMsData in"=w8) -> ("error out"=→"error out (DMMs) 2":errorcluster)  [unwired: 8 in, 1 out]
  n1327 = call-dynamic "USBData_terminate.vi"("error in (no error)"=w39, "USBData in"=w40) -> ("error out"=w41:errorcluster)  [unwired: 8 in, 1 out]
  n1328 = call-dynamic "LSI336Data_terminate.vi"("error in (no error)"=w30, "LSI336Data in"=w31) -> ("error out"=w29:errorcluster)  [unwired: 8 in, 1 out]
  n1329 = Merge Errors(w11, w13) -> (w14:errorcluster)
  n1330 = local write "error out (USB6210)"(w41) -> ()
  n1331 = local write "error out (LSI336)"(w29) -> ()
  n1332 = call "LSI218Data_terminate.vi"("error in (no error)"=w34, "LSI218Data in"=w35) -> ("error out"=w33:errorcluster)  [unwired: 8 in, 1 out]
  n1333 = Release Notifier(notifier=w12, error in (no error)=w14) -> (error out=→"error out (notifier)":errorcluster)  [unwired: 1 in, 2 out]
  n1334 = local write "error out (LSI218)"(w33) -> ()
